vi "UHR-Fleezers Control (host) - 10.6.vi"() -> ()   [LabVIEW 2010] (continued)
          }
        }
      }
      event "Inject Bottom": Value Change {
        n1712 = event-data() -> ("NewVal"=w7676:bool)  [unwired: 6 out]
        n1713 = disable-structure shown="Enabled" {
          disable-tunnel: w7678 -> [_ w7721]
          disable-tunnel: [_ w7720] -> w7677
          disable-tunnel: w7676 -> [_ w7719]
          frame Disabled {
            n1714 = local read "Pump write delay (ms)"() -> (w7680:dbl)
            n1715 = case shown="False" "Inject Bottom" {
              tunnel: w7680 -> [w7687 w7701]
              tunnel: "Chemyx Syringe Pump Serial Port" -> [w7684 w7700]
              frame False {
                n1716 = flat-sequence {
                  tunnel: w7684 -> [w7688]
                  tunnel: [w7688] -> w7685
                  tunnel: w7687 -> [_]
                  tunnel: [w7691] -> w7686
                  tunnel: w7685 -> [w7691]
                  tunnel: w7686 -> [w7692]
                  tunnel: [w7692] -> w7682
                  tunnel: [w7694] -> w7683
                  tunnel: w7682 -> [w7694]
                  tunnel: w7683 -> [w7696]
                  frame #0 {
                    n1717 = call "Write to pump.vi"("string"="enter pump3", "VISA resource name"=w7688) -> ()  [unwired: 1 out]
                  }
                  frame #1 {
                    n1718 = local read "Pump pause delay (ms)"() -> (w7690:u32)
                    n1719 = Wait (ms)(milliseconds to wait=w7690) -> ()  [unwired: 1 out]
                  }
                  frame #2 {
                    n1720 = call "Write to pump.vi"("string"="stop", "VISA resource name"=w7692) -> ()  [unwired: 1 out]
                  }
                  frame #3 {
                    n1721 = Wait (ms)(milliseconds to wait=u32 0) -> ()  [unwired: 1 out]
                  }
                  frame #4 {
                    n1722 = call "Write to pump.vi"("string"="stop", "VISA resource name"=w7696) -> ()  [unwired: 1 out]
                  }
                }
              }
              frame True {
                n1723 = flat-sequence {
                  tunnel: w7700 -> [w7710]
                  tunnel: w7701 -> [w7705]
                  tunnel: w7701 -> [w7712]
                  tunnel: w7700 -> [w7713]
                  tunnel: [w7713] -> w7698
                  tunnel: [w7716] -> w7699
                  tunnel: w7698 -> [w7716]
                  tunnel: w7699 -> [w7717]
                  frame #0 {
                    n1724 = local read "All Pump Parameters"() -> (w7704:T5)
                    n1725 = Unbundle By Name(w7704) -> ("Pump 3"=w7711:T51)
                    n1726 = call "Set pump parameters.vi"("Pump write delay (ms)"=w7705, "Volume (uL)"="Ch 3 Inject Volume (uL)", "Rate (uL/h)"="Ch 3 Inject Rate (ul/h)", "Units"=4.0, "Pump #"=3.0, "Pump Parameters In"=w7711, "VISA resource name"=w7710) -> ("Pump Parameters Out"=w7703:T51)  [unwired: 3 in]
                    n1727 = Bundle By Name(cluster=w7704, "Pump 3"=w7703) -> (w7702:T5)
                    n1728 = local write "All Pump Parameters"(w7702) -> ()
                  }
                  frame #1 {
                    n1729 = Wait (ms)(milliseconds to wait=w7712) -> ()  [unwired: 1 out]
                  }
                  frame #2 {
                    n1730 = call "Write to pump.vi"("string"="start", "VISA resource name"=w7713) -> ()  [unwired: 1 out]
                  }
                  frame #3 {
                    n1731 = Wait (ms)(milliseconds to wait=u32 500) -> ()  [unwired: 1 out]
                  }
                  frame #4 {
                    n1732 = call "Write to pump.vi"("string"="start", "VISA resource name"=w7717) -> ()  [unwired: 1 out]
                  }
                }
              }
            }
          }
          frame Enabled {
            n1733 = call "hamilton_controller.vi"("error in"=w7721, "Open?"=w7719, "valve"=enum16{"A", "B", "C", "D", "ALL"}."B", "action"=T17."MOVE VALVE") -> ("error out"=w7720:errorcluster)  [unwired: 7 in]
          }
        }
      }
      event "Inject Pump 2": Value Change {
        n1734 = event-data() -> ("NewVal"=w7724:bool)  [unwired: 6 out]
        n1735 = disable-structure shown="Enabled" {
          disable-tunnel: w7726 -> [_ w7749]
          disable-tunnel: [_ w7748] -> w7725
          disable-tunnel: w7724 -> [_ w7747]
          frame Disabled {
            n1736 = local read "Pump write delay (ms)"() -> (w7729:dbl)
            n1737 = flat-sequence {
              tunnel: w7727 -> [w7742]
              tunnel: w7729 -> [w7738]
              tunnel: "Inject Pump 2" -> [_]
              tunnel: w7729 -> [w7744]
              tunnel: w7727 -> [w7745]
              frame #0 {
                n1738 = local read "All Pump Parameters"() -> (w7737:T5)
                n1739 = Multiply(x=60.0, y="Flush Center Ch Rate (ul/m)") -> (x*y=w7734:dbl)
                n1740 = Unbundle By Name(w7737) -> ("Pump 2"=w7743:T51)
                n1741 = call "Set pump parameters.vi"("Pump write delay (ms)"=w7738, "Volume (uL)"="Flush Center Ch Volume (uL)", "Rate (uL/h)"=w7734, "Units"=3.0, "Pump #"=2.0, "Pump Parameters In"=w7743, "VISA resource name"=w7742) -> ("Pump Parameters Out"=w7736:T51)  [unwired: 3 in]
                n1742 = Bundle By Name(cluster=w7737, "Pump 2"=w7736) -> (w7735:T5)
                n1743 = local write "All Pump Parameters"(w7735) -> ()
                n1744 = Add(x="Flush Center Ch Volume (uL)", y="Total Volume\nFlushed (uL)") -> (x+y=w7731:dbl)
                n1745 = local write "Total Volume\nFlushed (uL)"(w7731) -> ()
              }
              frame #1 {
                n1746 = Wait (ms)(milliseconds to wait=w7744) -> ()  [unwired: 1 out]
              }
              frame #2 {
                n1747 = call "Write to pump.vi"("string"="start", "VISA resource name"=w7745) -> ()  [unwired: 1 out]
              }
            }
            n1748 = local read "Chemyx Syringe Pump Serial Port"() -> (w7727:refnum<visa-resource-name>)
          }
          frame Enabled {
            n1749 = call "hamilton_controller.vi"("error in"=w7749, "Open?"=w7747, "valve"=enum16{"A", "B", "C", "D", "ALL"}."B", "action"=T17."MOVE VALVE") -> ("error out"=w7748:errorcluster)  [unwired: 7 in]
          }
        }
      }
      event "Sample Channel Flow": Value Change {
        n1750 = event-data() -> ()  [unwired: 7 out]
        n1751 = call "hamilton_controller.vi"("error in"=w7753, "Open?"="Sample Channel Flow", "valve"=enum16{"A", "B", "C", "D", "ALL"}."C", "action"=T17."MOVE VALVE") -> ("error out"=w7752:errorcluster)  [unwired: 7 in]
      }
      event "Flip Green Filter": Value Change {
        n1752 = event-data() -> ()  [unwired: 7 out]
        n1753 = Not(x="Flip Green Filter") -> (.not. x?=w7757:bool)
        n1754 = local write "Flip Green Filter"(w7757) -> ()
        n1755 = flat-sequence {
          tunnel: w7765 -> [w7770]
          tunnel: w7764 -> [w7769]
          tunnel: [w7767] -> w7762
          tunnel: [w7766] -> w7761
          tunnel: [w7810] -> w7760
          tunnel: w7762 -> [w7810]
          tunnel: [w7809] -> w7759
          tunnel: w7761 -> [w7809]
          tunnel: w7760 -> [w7814]
          tunnel: w7759 -> [w7813]
          tunnel: [w7812] -> w7763
          frame #0 {
            n1756 = xnode "Read/Write Control"("FPGA VI Reference In"=w7770, "error in"=w7769, "Green Filter Flipper"=TRUE) -> ("FPGA VI Reference Out"=w7767:T20, "error out"=w7766:errorcluster)
          }
          frame #1 {
            n1757 = Wait (ms)(milliseconds to wait=u32 100) -> ()  [unwired: 1 out]
          }
          frame #2 {
            n1758 = xnode "Read/Write Control"("FPGA VI Reference In"=w7814, "error in"=w7813, "Green Filter Flipper"=FALSE) -> ("error out"=w7812:errorcluster)  [unwired: 1 out]
          }
        }
      }
      event "Pump 1 contents", "Pump 3 contents": Value Change {
        n1759 = event-data() -> ()  [unwired: 7 out]
        n1760 = local read "Pump 1 contents"() -> (→"Pump 1 cont disp":string)
        n1761 = local read "Pump 3 contents"() -> (→"Pump 3 cont disp":string)
      }
      event "Reset Trap Pos. FB": Value Change {
        n1762 = event-data() -> ()  [unwired: 7 out]
        n1763 = xnode "Read/Write Control"("FPGA VI Reference In"=w7858, "error in"=w7857, "Trap Pos. FB Reset"="Reset Trap Pos. FB") -> ()  [unwired: 2 out]
      }
      event "Trap Pos. FB ON": Value Change {
        n1764 = event-data() -> ()  [unwired: 7 out]
        n1765 = xnode "Read/Write Control"("FPGA VI Reference In"=w7899, "error in"=w7898, "Force feedback"="Trap Pos. FB ON") -> ()  [unwired: 2 out]
      }
      event "Trap Pos. FB Range", "Trap Pos. FB Gains", "Trap Pos. FB Mult Factor", "Trap Pos. FB Offset Factor", "Trap Pos FB Negate Action", "Trap Pos FB Monitor\nT1 or T2": Value Change {
        n1766 = event-data() -> ()  [unwired: 7 out]
        n1767 = xnode "Read/Write Control"("FPGA VI Reference In"=w7946, "error in"=w7945, "Trap Pos. FB Range"="Trap Pos. FB Range", "Trap Pos. FB Gains"="Trap Pos. FB Gains", "Trap Pos. FB Mult Factor"="Trap Pos. FB Mult Factor", "Trap Pos. FB Offset Factor"="Trap Pos. FB Offset Factor", "Trap Pos FB Negate Action"="Trap Pos FB Negate Action", "Trap Pos FB Monitor T1 or T2"="Trap Pos FB Monitor\nT1 or T2", "AI1 X Scale"="Trap Pos. AI1 X Pre-scale") -> ()  [unwired: 2 out]
      }
      event "Trap Pos FB SP": Value Change {
        n1768 = event-data() -> ()  [unwired: 7 out]
        n1769 = xnode "Read/Write Control"("FPGA VI Reference In"=w8134, "error in"=w8133, "Trap Pos. FB SP"="Trap Pos FB SP") -> ()  [unwired: 2 out]
      }
      event "Set SP to Reading": Value Change {
        n1770 = event-data() -> ()  [unwired: 7 out]
        n1771 = local read "Trap Pos FB Monitor\nT1 or T2"() -> (w8187:bool)
        n1772 = local read "Trap X AI1 (DMA)"() -> (w8190:T13)
        n1773 = local read "Trap X (AI1)"() -> (w8193:T10)
        n1774 = Unbundle By Name(w8193) -> ("Trap 1"=w8192:fxp<+/-,16,1>, "Trap 2"=w8191:fxp<+/-,16,1>)
        n1775 = Unbundle By Name(w8190) -> ("Set 1"=w8189:fxp<+/-,16,1>, "Set 2"=w8188:fxp<+/-,16,1>)
        n1776 = Select(t=w8192, s=w8187, f=w8191) -> (s? t:f=w8186:fxp<+/-,16,1>)
        n1777 = Select(t=w8189, s=w8187, f=w8188) -> (s? t:f=w8185:fxp<+/-,16,1>)
        n1778 = Not(x="Set SP Using...") -> (.not. x?=w8180:bool)
        n1779 = Select(t=w8186, s=w8180, f=w8185) -> (s? t:f=w8181:fxp<+/-,16,1>)
        n1780 = xnode "Read/Write Control"("FPGA VI Reference In"=w8183, "error in"=w8182, "Trap Pos. FB SP"=w8181) -> ()  [unwired: 2 out]
        n1781 = local write "Trap Pos FB SP"(w8181) -> ()
      }
      event "Trap Pos. FB Out Scale 2^n": Value Change {
        n1782 = event-data() -> ()  [unwired: 7 out]
        n1783 = Scale By Power Of 2(n="Trap Pos. FB Out Scale 2^n", x=ext 1.0) -> (x*2^n=w8240:ext)
        n1784 = property on="Trap Pos. FB Mult Factor" class="DigNum (strict)"("Val(Sgnl)"=w8240) -> ()  [unwired: 2 in, 2 out]
      }
      event "Trap Pos FB Int Count": Value Change {
        n1785 = event-data() -> ()  [unwired: 7 out]
        n1786 = xnode "Read/Write Control"("FPGA VI Reference In"=w8245, "error in"=w8244, "Trap Pos FB Int Count"="Trap Pos FB Int Count") -> ()  [unwired: 2 out]
      }
    }
    "error out 2" <- w4492
    n1787 = node-c288() -> ()  [unwired: 1 in, 1 out]
  }
  n1788 = timed-loop "Run Scripts, including: stage motion" {
    timing: w74 -> [_]
    timing-out: [_] -> w73
    tunnel: w18 -> [_]
    stop <- w8284 stop-if-true
    n1789 = node-c288() -> ()  [unwired: 1 in, 1 out]
    n1790 = event shown="[15] \"Take Detection Laser\nImage\": Value Change" {
      selector: _ -> [_ _ _ _ _ _ _ _ _ _ _ _ _ _ _ _ _]
      dyn-events: _ -> [_ _ _ _ _ _ _ _ _ _ _ _ _ _ _ _ _]
      timeout: 50 -> [_ _ _ _ _ _ _ _ _ _ _ _ _ _ _ _ _]
      tunnel: ["Set Position" "Move to Position" "Move Cap. 1 (DNA Right)" _ "Move Cap. 2 (ADig Left)" _ "Cal/Data Acq. Spot" "Dump Beads" "Dip for Protein" _ _ "Got ADig bead" "Got DNA bead" "Take Stepping Data" _ "Take Detection Laser\nImage" _] -> _
      tunnel: [_ _ _ _ _ _ _ _ _ _ _ _ _ _ _ _ w8671] -> w8284
      event "Set Position", "Set Position 2", "Set Position 3", "Set Position 4", "Set Position 5", "Set Position 1": Value Change {
        n1791 = event-data() -> ()  [unwired: 1 in, 5 out]
        n1792 = Build Array("Set Position 1", "Set Position 2", "Set Position 3", "Set Position 4", "Set Position 5") -> (w8303:bool[])
        n1793 = Boolean Array To Number(Boolean array=w8303) -> (number=w8302:u32)
        n1794 = Logarithm Base 2(1:w8302) -> (0:w8294:dbl)
        n1795 = call "CONEX_FUNCTIONAL_GLOBAL.vi"("Command"=T23."GET POS") -> ("Current Position"=w8287:dbl[])  [unwired: 8 in, 2 out]
        n1796 = Decrement(x="Position") -> (x-1=w8292:dbl)
        n1797 = Greater Or Equal?(x=w8294, y=0.0) -> (x >= y?=w8295:bool)
        n1798 = Select(t=w8294, s=w8295, f=w8292) -> (s? t:f=w8291:dbl)
        n1799 = Increment(x=w8291) -> (x+1=w8290:dbl)
        n1800 = Build Array (concatenate)(w8290, w8287) -> (w8289:dbl[])
        n1801 = Replace Array Subset(array="Saved Stage Positions", new element=w8289, index (row)=w8291) -> (w8304:dbl[][])  [unwired: 1 in]
        n1802 = local write "Saved Stage Positions"(w8304) -> ()
      }
      event "Move to Position": Value Change {
        n1803 = event-data() -> ()  [unwired: 1 in, 5 out]
        n1804 = flat-sequence {
          frame #0 {
            n1805 = local read "Position"() -> (w8319:dbl)
            n1806 = local read "Saved Stage Positions"() -> (w8317:dbl[][])
            n1807 = Decrement(x=w8319) -> (x-1=w8316:dbl)
            n1808 = Array Subset(array=w8317, index (row)=w8316, length (row)=1 ("length"), index (col)=1 ("index"), length (col)=3 ("length")) -> (w8313:dbl[][])
            n1809 = Reshape Array(w8313, 3 ("dimension size")) -> (w8309:dbl[])
            n1810 = local write "Stage Moving"(TRUE ("Stage Moving")) -> ()
            n1811 = call "CONEX_FUNCTIONAL_GLOBAL.vi"("Axis"=enum16{"X", "Y", "Z", "XY", "XZ", "YZ", "XYZ"}."XYZ", "Position"=w8309, "Command"=T23."ABS MOVE") -> ()  [unwired: 6 in, 3 out]
          }
          frame #1 {
            n1812 = call <vilib>:"Beep.vi"() -> ()  [unwired: 3 in, 9 out]
            n1813 = local write "Stage Moving"(FALSE ("Stage Moving")) -> ()
          }
        }
      }
      event "Move Cap. 1 (DNA Right)": Value Change {
        n1814 = event-data() -> ()  [unwired: 1 in, 5 out]
        n1815 = local write "Move Cap. 1 (DNA Right)"(FALSE ("Move Cap. 1 (DNA Right)")) -> ()
        n1816 = flat-sequence {
          tunnel: ["Cap 1 Samp Flow ON"] -> w8322
          tunnel: w8322 -> [w8341]
          tunnel: [w8341] -> w8321
          tunnel: w8321 -> [w8342]
          frame #0 {
            n1817 = local read "Saved Stage Positions"() -> (w8335:dbl[][])
            n1818 = Array Subset(array=w8335, index (row)=0 ("index"), length (row)=1 ("length"), index (col)=1 ("index"), length (col)=3 ("length")) -> (w8332:dbl[][])
            n1819 = Reshape Array(w8332, 3 ("dimension size")) -> (w8326:dbl[])
            n1820 = case shown="True" "Cap 1 Samp Flow ON" {
              frame False {
              }
              frame True {
                n1821 = call "hamilton_controller.vi"("Open?"=TRUE, "valve"=enum16{"A", "B", "C", "D", "ALL"}."C", "action"=T17."MOVE VALVE") -> ()  [unwired: 8 in, 1 out]
              }
            }
            n1822 = call "CONEX_FUNCTIONAL_GLOBAL.vi"("Axis"=enum16{"X", "Y", "Z", "XY", "XZ", "YZ", "XYZ"}."XYZ", "Position"=w8326, "Command"=T23."ABS MOVE") -> ()  [unwired: 6 in, 3 out]
            n1823 = local write "Stage Moving"(TRUE ("Stage Moving")) -> ()
          }
          frame #1 {
            n1824 = call "motor_done_moving.vi"("wait at least (s)"=2.0) -> ()  [unwired: 11 in]
          }
          frame #2 {
            n1825 = local write "Stage Moving"(FALSE ("Stage Moving")) -> ()
            n1826 = case shown="True" w8342 {
              frame False {
              }
              frame True {
                n1827 = call "hamilton_controller.vi"("Open?"=FALSE, "valve"=enum16{"A", "B", "C", "D", "ALL"}."C", "action"=T17."MOVE VALVE") -> ()  [unwired: 8 in, 1 out]
              }
            }
            n1828 = case shown="True" TRUE {
              tunnel: "Cap 1 T ON" -> [w8351 w8352]
              frame False {
                n1829 = property on="Trap 1 (ON/OFF)" class="Bool (strict)"("Val(Sgnl)"=w8351) -> ()  [unwired: 2 in, 2 out]
              }
              frame True {
                n1830 = property on="Trap 2 (ON/OFF)" class="Bool (strict)"("Val(Sgnl)"=w8352) -> ()  [unwired: 2 in, 2 out]
              }
            }
            n1831 = call <vilib>:"Beep.vi"() -> ()  [unwired: 3 in, 9 out]
            n1832 = case shown="True" "Cap 1 Flow ON" {
              frame False {
              }
              frame True {
                n1833 = property on="Inject Top" class="Bool (strict)"("Val(Sgnl)"=TRUE ("Value (Signaling)")) -> ()  [unwired: 2 in, 2 out]
              }
            }
          }
        }
      }
      event Timeout {
        n1834 = event-data() -> ()  [unwired: 1 in, 2 out]
      }
      event "Move Cap. 2 (ADig Left)": Value Change {
        n1835 = event-data() -> ()  [unwired: 1 in, 5 out]
        n1836 = local write "Move Cap. 2 (ADig Left)"(FALSE ("Move Cap. 2 (ADig Left)")) -> ()
        n1837 = flat-sequence {
          tunnel: ["Cap 2 Samp Flow ON"] -> w8354
          tunnel: w8354 -> [w8373]
          tunnel: [w8373] -> w8353
          tunnel: w8353 -> [w8374]
          frame #0 {
            n1838 = local read "Saved Stage Positions"() -> (w8367:dbl[][])
            n1839 = case shown="True" "Cap 2 Samp Flow ON" {
              frame False {
              }
              frame True {
                n1840 = call "hamilton_controller.vi"("Open?"=TRUE, "valve"=enum16{"A", "B", "C", "D", "ALL"}."C", "action"=T17."MOVE VALVE") -> ()  [unwired: 8 in, 1 out]
              }
            }
            n1841 = Array Subset(array=w8367, index (row)=1 ("index"), length (row)=1 ("length"), index (col)=1 ("index"), length (col)=3 ("length")) -> (w8364:dbl[][])
            n1842 = Reshape Array(w8364, 3 ("dimension size")) -> (w8358:dbl[])
            n1843 = local write "Stage Moving"(TRUE ("Stage Moving")) -> ()
            n1844 = call "CONEX_FUNCTIONAL_GLOBAL.vi"("Axis"=enum16{"X", "Y", "Z", "XY", "XZ", "YZ", "XYZ"}."XYZ", "Position"=w8358, "Command"=T23."ABS MOVE") -> ()  [unwired: 6 in, 3 out]
          }
          frame #1 {
            n1845 = call "motor_done_moving.vi"("wait at least (s)"=2.0) -> ()  [unwired: 11 in]
          }
          frame #2 {
            n1846 = local write "Stage Moving"(FALSE ("Stage Moving")) -> ()
            n1847 = case shown="True" TRUE {
              tunnel: "Cap 2 T ON" -> [w8383 w8384]
              frame False {
                n1848 = property on="Trap 2 (ON/OFF)" class="Bool (strict)"("Val(Sgnl)"=w8383) -> ()  [unwired: 2 in, 2 out]
              }
              frame True {
                n1849 = property on="Trap 1 (ON/OFF)" class="Bool (strict)"("Val(Sgnl)"=w8384) -> ()  [unwired: 2 in, 2 out]
              }
            }
            n1850 = call <vilib>:"Beep.vi"() -> ()  [unwired: 3 in, 9 out]
            n1851 = case shown="True" w8374 {
              frame False {
              }
              frame True {
                n1852 = call "hamilton_controller.vi"("Open?"=FALSE, "valve"=enum16{"A", "B", "C", "D", "ALL"}."C", "action"=T17."MOVE VALVE") -> ()  [unwired: 8 in, 1 out]
              }
            }
            n1853 = case shown="True" "Cap 2 Flow ON" {
              frame False {
              }
              frame True {
                n1854 = property on="Inject Bottom" class="Bool (strict)"("Val(Sgnl)"=TRUE ("Value (Signaling)")) -> ()  [unwired: 2 in, 2 out]
              }
            }
          }
        }
      }
      event "+z", "-z": Value Change {
        n1855 = event-data() -> ()  [unwired: 1 in, 5 out]
        n1856 = flat-sequence {
          frame #0 {
            w8386 = 0.0 ("element")
            n1857 = Divide(x="z nudge increment (um)", y=1000.0) -> (x/y=w8399:dbl)
            n1858 = Boolean To (0,1)(Boolean="+z") -> (0, 1=w8392:i16)
            n1859 = Boolean To (0,1)(Boolean="-z") -> (0, 1=w8393:i16)
            n1860 = Multiply(x=w8392, y=w8399) -> (x*y=w8396:dbl)
            n1861 = Multiply(x=w8393, y=w8399) -> (x*y=w8394:dbl)
            n1862 = Negate(x=w8394) -> (-x=w8395:dbl)
            n1863 = Add(x=w8396, y=w8395) -> (x+y=w8387:dbl)
            n1864 = Build Array(w8386, w8386, w8387) -> (w8385:dbl[])
            n1865 = call "CONEX_FUNCTIONAL_GLOBAL.vi"("Axis"=enum16{"X", "Y", "Z", "XY", "XZ", "YZ", "XYZ"}."Z", "Position"=w8385, "Command"=T23."REL MOVE") -> ()  [unwired: 6 in, 3 out]
            n1866 = local write "Stage Moving"(TRUE ("Stage Moving")) -> ()
          }
          frame #1 {
            n1867 = local write "Stage Moving"(FALSE ("Stage Moving")) -> ()
            n1868 = call <vilib>:"Beep.vi"() -> ()  [unwired: 3 in, 9 out]
          }
        }
      }
      event "Cal/Data Acq. Spot": Value Change {
        # "CHANGE FISH FOR TETHER BACK\nTO TRUE VALUE HERE."
        n1869 = event-data() -> ()  [unwired: 1 in, 5 out]
        n1870 = flat-sequence {
          tunnel: ["Cal @ (MHz)"] -> w8402
          tunnel: w8402 -> [w8425]
          tunnel: w8402 -> [w8446]
          frame #0 {
            n1871 = local read "Saved Stage Positions"() -> (w8410:dbl[][])
            n1872 = Array Subset(array=w8410, index (row)=2 ("index"), length (row)=1 ("length"), index (col)=1 ("index"), length (col)=3 ("length")) -> (w8413:dbl[][])
            n1873 = Reshape Array(w8413, 3 ("dimension size")) -> (w8406:dbl[])
            n1874 = local write "Stage Moving"(TRUE ("Stage Moving")) -> ()
            n1875 = call "CONEX_FUNCTIONAL_GLOBAL.vi"("Axis"=enum16{"X", "Y", "Z", "XY", "XZ", "YZ", "XYZ"}."XYZ", "Position"=w8406, "Command"=T23."ABS MOVE") -> ()  [unwired: 6 in, 3 out]
          }
          frame #1 {
            n1876 = call "motor_done_moving.vi"("wait at least (s)"=2.0) -> ()  [unwired: 11 in]
          }
          frame #2 {
            n1877 = property on="Trap Delta (MHz)" class="DigNum (strict)"("Val(Sgnl)"="Cal @ (MHz)") -> ()  [unwired: 2 in, 2 out]
            n1878 = local write "Stage Moving"(FALSE ("Stage Moving")) -> ()
            n1879 = call <vilib>:"Beep.vi"() -> ()  [unwired: 3 in, 9 out]
          }
          frame #3 {
            n1880 = Wait (ms)(milliseconds to wait=u32 100) -> ()  [unwired: 1 out]
          }
          frame #4 {
            n1881 = property on="Save Calibration" class="Bool (strict)"("Val(Sgnl)"=TRUE ("Value (Signaling)")) -> ()  [unwired: 2 in, 2 out]
          }
          frame #5 {
            n1882 = Wait (ms)(milliseconds to wait=u32 4000) -> ()  [unwired: 1 out]
          }
          frame #6 {
            n1883 = while {
              stop <- w8422 stop-if-true
              n1884 = local read "Saving..."() -> (w8423:bool)
              n1885 = Wait (ms)(milliseconds to wait=u32 100) -> ()  [unwired: 1 out]
              n1886 = Not(x=w8423) -> (.not. x?=w8422:bool)
            }
          }
          frame #7 {
            n1887 = case shown="True" "W/ Offset 1" {
              tunnel: w8425 -> [_ w8427]
              frame False {
              }
              frame True {
                n1888 = stacked-sequence {
                  tunnel: w8427 -> [_ _ _ _ _ _ _ w8444]
                  frame #0 {
                    n1889 = property on="Trap Delta (MHz)" class="DigNum (strict)"("Val(Sgnl)"="Offset 1 Start (MHz)") -> ()  [unwired: 2 in, 2 out]
                    n1890 = Replace Array Subset(array=u32[] [0] ("Index Values"), new element="Offset 1 Set", index=0) -> (w8428:u32[])
                    n1891 = property on="Saved AOD Raster Scan Parameter Sets" class="Arr (strict)"("Index Values"=w8428) -> ()  [unwired: 2 in, 2 out]
                  }
                  frame #1 {
                    n1892 = Wait (ms)(milliseconds to wait=u32 200) -> ()  [unwired: 1 out]
                  }
                  frame #2 {
                    n1893 = property on="Load parameters" class="Bool (strict)"("Val(Sgnl)"=TRUE ("Value (Signaling)")) -> ()  [unwired: 2 in, 2 out]
                  }
                  frame #3 {
                    n1894 = Wait (ms)(milliseconds to wait=u32 200) -> ()  [unwired: 1 out]
                  }
                  frame #4 {
                    n1895 = property on="Trap Raster Scan" class="Bool (strict)"("Val(Sgnl)"=TRUE ("Value (Signaling)")) -> ()  [unwired: 2 in, 2 out]
                  }
                  frame #5 {
                    n1896 = Wait (ms)(milliseconds to wait=u32 2000) -> ()  [unwired: 1 out]
                  }
                  frame #6 {
                    n1897 = while {
                      stop <- w8441 stop-if-true
                      n1898 = local read "Raster Scanning..."() -> (w8443:bool)
                      n1899 = local read "Saving..."() -> (w8439:bool)
                      n1900 = Wait (ms)(milliseconds to wait=u32 100) -> ()  [unwired: 1 out]
                      n1901 = Not(x=w8439) -> (.not. x?=w8438:bool)
                      n1902 = Not(x=w8443) -> (.not. x?=w8440:bool)
                      n1903 = And(x=w8440, y=w8438) -> (x .and. y?=w8441:bool)
                    }
                  }
                  frame #7 {
                    n1904 = property on="Trap Delta (MHz)" class="DigNum (strict)"("Val(Sgnl)"=w8444) -> ()  [unwired: 2 in, 2 out]
                  }
                }
              }
            }
          }
          frame #8 {
            n1905 = local read "Save ave N"() -> (w8445:dbl)
            n1906 = case shown="True" "W/ Offset 2" {
              tunnel: w8446 -> [_ w8452]
              tunnel: w8445 -> [_ w8451]
              frame False {
                n1907 = Multiply(x="Cal read wait (s)", y=u32 1000 ("milliseconds to wait")) -> (x*y=w8449:u32)
                n1908 = Wait (ms)(milliseconds to wait=w8449) -> ()  [unwired: 1 out]
              }
              frame True {
                n1909 = stacked-sequence {
                  tunnel: w8452 -> [_ _ _ _ _ _ _ _ _ w8473 _ _]
                  tunnel: w8451 -> [_ _ _ _ _ _ _ _ _ w8471 _ _]
                  frame #0 {
                    n1910 = property on="Save ave N" class="DigNum (strict)"("Val(Sgnl)"=1.0 ("Value (Signaling)")) -> ()  [unwired: 2 in, 2 out]
                  }
                  frame #1 {
                    n1911 = Wait (ms)(milliseconds to wait=u32 500) -> ()  [unwired: 1 out]
                  }
                  frame #2 {
                    n1912 = property on="Trap Delta (MHz)" class="DigNum (strict)"("Val(Sgnl)"="Offset 2 Start (MHz)") -> ()  [unwired: 2 in, 2 out]
                    n1913 = Replace Array Subset(array=u32[] [0] ("Index Values"), new element="Offset 2 Set", index=0) -> (w8457:u32[])
                    n1914 = property on="Saved AOD Raster Scan Parameter Sets" class="Arr (strict)"("Index Values"=w8457) -> ()  [unwired: 2 in, 2 out]
                  }
                  frame #3 {
                    n1915 = Wait (ms)(milliseconds to wait=u32 500) -> ()  [unwired: 1 out]
                  }
                  frame #4 {
                    n1916 = property on="Load parameters" class="Bool (strict)"("Val(Sgnl)"=TRUE ("Value (Signaling)")) -> ()  [unwired: 2 in, 2 out]
                  }
                  frame #5 {
                    n1917 = Wait (ms)(milliseconds to wait=u32 500) -> ()  [unwired: 1 out]
                  }
                  frame #6 {
                    n1918 = property on="Trap Raster Scan" class="Bool (strict)"("Val(Sgnl)"=TRUE ("Value (Signaling)")) -> ()  [unwired: 2 in, 2 out]
                  }
                  frame #7 {
                    n1919 = Wait (ms)(milliseconds to wait=u32 2000) -> ()  [unwired: 1 out]
                  }
                  frame #8 {
                    n1920 = while {
                      stop <- w8466 stop-if-true
                      n1921 = local read "Raster Scanning..."() -> (w8469:bool)
                      n1922 = local read "Saving..."() -> (w8467:bool)
                      n1923 = Wait (ms)(milliseconds to wait=u32 100) -> ()  [unwired: 1 out]
                      n1924 = Not(x=w8467) -> (.not. x?=w8465:bool)
                      n1925 = Not(x=w8469) -> (.not. x?=w8468:bool)
                      n1926 = And(x=w8468, y=w8465) -> (x .and. y?=w8466:bool)
                    }
                  }
                  frame #9 {
                    n1927 = property on="Trap Delta (MHz)" class="DigNum (strict)"("Val(Sgnl)"=w8473) -> ()  [unwired: 2 in, 2 out]
                    n1928 = property on="Saved AOD Raster Scan Parameter Sets" class="Arr (strict)"("Index Values"=u32[] [0]) -> ()  [unwired: 2 in, 2 out]
                    n1929 = property on="Save ave N" class="DigNum (strict)"("Val(Sgnl)"=w8471) -> ()  [unwired: 2 in, 2 out]
                  }
                  frame #10 {
                    n1930 = Wait (ms)(milliseconds to wait=u32 500) -> ()  [unwired: 1 out]
                  }
                  frame #11 {
                    n1931 = property on="Load parameters" class="Bool (strict)"("Val(Sgnl)"=TRUE ("Value (Signaling)")) -> ()  [unwired: 2 in, 2 out]
                  }
                }
              }
            }
          }
          frame #9 {
            n1932 = property on="Read Cal" class="Bool (strict)"("Val(Sgnl)"=TRUE ("Value (Signaling)")) -> ()  [unwired: 2 in, 2 out]
          }
          frame #10 {
            n1933 = Wait (ms)(milliseconds to wait=u32 500) -> ()  [unwired: 1 out]
          }
          frame #11 {
            n1934 = property on="Fish for Tether" class="Bool (strict)"("Val(Sgnl)"="fish after calibration?") -> ()  [unwired: 2 in, 2 out]
          }
        }
        n1935 = local write "Cal/Data Acq. Spot"(FALSE ("Cal/Data Acq. Spot")) -> ()
      }
      event "Dump Beads": Value Change {
        # "SCRIPT TO REMOVE BOTH BEADS FROM THE TRAPS. TURNS ON LIGHT WHICH INDICATES THAT STAGE IS MOVING. THEN STOPS SAVING DATA. \nSETS Sample Channel Flow TO TRUE. STOPS INTERLACING GREEN FLUORESCENCE. TURNS OFF Tether INDICATOR BECAUSE WE ARE THROWING IT\nAWAY. SHUTS OFF TRAP POSITION FEEDBACK."
        n1936 = event-data() -> ()  [unwired: 1 in, 5 out]
        n1937 = flat-sequence {
          frame #0 {
            w8481 = FALSE ("Fl. Triggered...")
            w8480 = TRUE ("Stage Moving")
            n1938 = local read "Saving..."() -> (w8482:bool)
            n1939 = local write "Fl. Triggered..."(w8481) -> ()
            n1940 = local write "Stage Moving"(w8480) -> ()
            n1941 = local write "Tether"(w8481) -> ()
            n1942 = property on="Green Laser ON/Interlacing" class="Bool (strict)"("Val(Sgnl)"=w8481) -> ()  [unwired: 2 in, 2 out]
            n1943 = property on="Trap Pos. FB ON" class="Bool (strict)"("Val(Sgnl)"=w8481) -> ()  [unwired: 2 in, 2 out]
            n1944 = property on="Sample Channel Flow" class="Bool (strict)"("Val(Sgnl)"=w8480) -> ()  [unwired: 2 in, 2 out]
            n1945 = local write "Stop Saving"(w8482) -> ()
          }
          frame #1 {
            # "MOVES TO THE DUMP BEADS POSITION"
            n1946 = local read "Saved Stage Positions"() -> (w8486:dbl[][])
            n1947 = Array Subset(array=w8486, index (row)=3 ("index"), length (row)=1 ("length"), index (col)=1 ("index"), length (col)=3 ("length")) -> (w8489:dbl[][])
            n1948 = Reshape Array(w8489, 3 ("dimension size")) -> (w8484:dbl[])
            n1949 = call "CONEX_FUNCTIONAL_GLOBAL.vi"("Axis"=enum16{"X", "Y", "Z", "XY", "XZ", "YZ", "XYZ"}."XYZ", "Position"=w8484, "Command"=T23."ABS MOVE") -> ()  [unwired: 6 in, 3 out]
          }
          frame #2 {
            n1950 = call "motor_done_moving.vi"("wait at least (s)"=2.0) -> ()  [unwired: 11 in]
          }
          frame #3 {
            w8494 = FALSE ("Value (Signaling)")
            # "TURNS TRAPS OFF SO THAT\nBEADS REMAIN AT DUMP \nBEADS POSITION"
            n1951 = property on="Trap 1 (ON/OFF)" class="Bool (strict)"("Val(Sgnl)"=w8494) -> ()  [unwired: 2 in, 2 out]
            n1952 = property on="Trap 2 (ON/OFF)" class="Bool (strict)"("Val(Sgnl)"=w8494) -> ()  [unwired: 2 in, 2 out]
            n1953 = call <vilib>:"Beep.vi"() -> ()  [unwired: 3 in, 9 out]
          }
          frame #4 {
            # "MOVES STAGE BACK TO THE\nANTIDIG CAPILARY BY CALLING\nTHE Move Cap. 2 SCRIPT"
            n1954 = property on="Move Cap. 2 (ADig Left)" class="Bool (strict)"("Val(Sgnl)"=TRUE ("Value (Signaling)")) -> ()  [unwired: 2 in, 2 out]
          }
        }
      }
      event "Dip for Protein": Value Change {
        n1955 = event-data() -> ()  [unwired: 1 in, 5 out]
        n1956 = flat-sequence {
          frame #0 {
            n1957 = case shown="True" "Move Trap Before?" {
              frame False {
              }
              frame True {
                n1958 = property on="Trap Delta (MHz)" class="DigNum (strict)"("Val(Sgnl)"="Dip Trap Delta 1 (MHz)") -> ()  [unwired: 2 in, 2 out]
              }
            }
          }
          frame #1 {
            n1959 = local read "Saved Stage Positions"() -> (w8502:dbl[][])
            n1960 = Array Subset(array=w8502, index (row)=4 ("index"), length (row)=1 ("length"), index (col)=1 ("index"), length (col)=3 ("length")) -> (w8505:dbl[][])
            n1961 = Reshape Array(w8505, 3 ("dimension size")) -> (w8500:dbl[])
            n1962 = call "CONEX_FUNCTIONAL_GLOBAL.vi"("Axis"=enum16{"X", "Y", "Z", "XY", "XZ", "YZ", "XYZ"}."XYZ", "Position"=w8500, "Command"=T23."ABS MOVE") -> ()  [unwired: 6 in, 3 out]
          }
          frame #2 {
            n1963 = Multiply(x="Duration (s)", y=1000.0) -> (x*y=w8509:dbl)
            n1964 = Wait (ms)(milliseconds to wait=w8509) -> ()  [unwired: 1 out]
          }
          frame #3 {
            n1965 = local read "Saved Stage Positions"() -> (w8515:dbl[][])
            n1966 = Array Subset(array=w8515, index (row)=2 ("index"), length (row)=1 ("length"), index (col)=1 ("index"), length (col)=3 ("length")) -> (w8518:dbl[][])
            n1967 = Reshape Array(w8518, 3 ("dimension size")) -> (w8513:dbl[])
            n1968 = call "CONEX_FUNCTIONAL_GLOBAL.vi"("Axis"=enum16{"X", "Y", "Z", "XY", "XZ", "YZ", "XYZ"}."XYZ", "Position"=w8513, "Command"=T23."ABS MOVE") -> ()  [unwired: 6 in, 3 out]
          }
          frame #4 {
            n1969 = case shown="True" "Move Trap After?" {
              frame False {
              }
              frame True {
                n1970 = property on="Trap Delta (MHz)" class="DigNum (strict)"("Val(Sgnl)"="Dip Trap Delta 2 (MHz)") -> ()  [unwired: 2 in, 2 out]
              }
            }
          }
          frame #5 {
            n1971 = case shown="True" "Green ON After?" {
              frame False {
              }
              frame True {
                n1972 = property on="Green Laser ON/Interlacing" class="Bool (strict)"("Val(Sgnl)"=TRUE ("Value (Signaling)")) -> ()  [unwired: 2 in, 2 out]
              }
            }
          }
          frame #6 {
            n1973 = Wait (ms)(milliseconds to wait=u32 500) -> ()  [unwired: 1 out]
          }
          frame #7 {
            n1974 = case shown="True" "Save Data After?" {
              frame False {
              }
              frame True {
                n1975 = property on="Start Saving" class="Bool (strict)"("Val(Sgnl)"=TRUE ("Value (Signaling)")) -> ()  [unwired: 2 in, 2 out]
              }
            }
          }
        }
      }
      event "Profile": Value Change {
        n1976 = event-data() -> ()  [unwired: 1 in, 5 out]
        n1977 = flat-sequence {
          tunnel: [w8531] -> w8530
          tunnel: w8530 -> [w8535]
          tunnel: [w8534] -> w8529
          tunnel: w8529 -> [w8541]
          frame #0 {
            w8532 = 0.0 ("element")
            n1978 = Build Array(w8532, "Y change (mm)", w8532) -> (w8531:dbl[])
          }
          frame #1 {
            # "move to new position and start saving"
            n1979 = local write "Stage Moving"(TRUE ("Stage Moving")) -> ()
            n1980 = local write "Start Saving"(TRUE ("Start Saving")) -> ()
            n1981 = call "CONEX_FUNCTIONAL_GLOBAL.vi"("Axis"=enum16{"X", "Y", "Z", "XY", "XZ", "YZ", "XYZ"}."Y", "Position"=w8535, "Command"=T23."REL MOVE") -> ()  [unwired: 6 in, 3 out]
            n1982 = Negate(x=w8535) -> (-x=w8534:dbl[])
          }
          frame #2 {
            # "go back to start"
            n1983 = call "CONEX_FUNCTIONAL_GLOBAL.vi"("Axis"=enum16{"X", "Y", "Z", "XY", "XZ", "YZ", "XYZ"}."Y", "Position"=w8541, "Command"=T23."REL MOVE") -> ()  [unwired: 6 in, 3 out]
          }
          frame #3 {
            # "stop saving"
            n1984 = local write "Stop Saving"(TRUE ("Stop Saving")) -> ()
            n1985 = local write "Stage Moving"(FALSE ("Stage Moving")) -> ()
          }
        }
      }
      event "Move to Position 1", "Move to Position 2", "Move to Position 3", "Move to Position 4", "Move to Position 5", "Lower Ch. Cap.": Value Change {
        n1986 = event-data() -> ()  [unwired: 1 in, 5 out]
        n1987 = Or(x="Move to Position 5", y="Lower Ch. Cap.") -> (x .or. y?=w8546:bool)
        n1988 = Build Array("Move to Position 1", "Move to Position 2", "Move to Position 3", "Move to Position 4", w8546) -> (w8549:bool[])
        n1989 = Boolean Array To Number(Boolean array=w8549) -> (number=w8548:u32)
        n1990 = Logarithm Base 2(1:w8548) -> (0:w8547:dbl)
        n1991 = flat-sequence {
          tunnel: w8547 -> [w8559]
          frame #0 {
            n1992 = local read "Saved Stage Positions"() -> (w8564:dbl[][])
            n1993 = Array Subset(array=w8564, index (row)=w8559, length (row)=1 ("length"), index (col)=1 ("index"), length (col)=3 ("length")) -> (w8561:dbl[][])
            n1994 = Reshape Array(w8561, 3 ("dimension size")) -> (w8556:dbl[])
            n1995 = local write "Stage Moving"(TRUE ("Stage Moving")) -> ()
            n1996 = call "CONEX_FUNCTIONAL_GLOBAL.vi"("Axis"=enum16{"X", "Y", "Z", "XY", "XZ", "YZ", "XYZ"}."XYZ", "Position"=w8556, "Command"=T23."ABS MOVE") -> ()  [unwired: 6 in, 3 out]
          }
          frame #1 {
            n1997 = local write "Stage Moving"(FALSE ("Stage Moving")) -> ()
            n1998 = call <vilib>:"Beep.vi"() -> ()  [unwired: 3 in, 9 out]
          }
        }
      }
      event "Got ADig bead": Value Change {
        n1999 = event-data() -> ()  [unwired: 1 in, 5 out]
        n2000 = property on="Move Cap. 1 (DNA Right)" class="Bool (strict)"("Val(Sgnl)"=TRUE ("Value (Signaling)")) -> ()  [unwired: 2 in, 2 out]
        n2001 = property on="Inject Bottom" class="Bool (strict)"("Val(Sgnl)"=FALSE ("Value (Signaling)")) -> ()  [unwired: 2 in, 2 out]
      }
      event "Got DNA bead": Value Change {
        n2002 = event-data() -> ()  [unwired: 1 in, 5 out]
        n2003 = property on="Cal/Data Acq. Spot" class="Bool (strict)"("Val(Sgnl)"=TRUE ("Value (Signaling)")) -> ()  [unwired: 2 in, 2 out]
        n2004 = property on="Inject Top" class="Bool (strict)"("Val(Sgnl)"=FALSE ("Value (Signaling)")) -> ()  [unwired: 2 in, 2 out]
      }
      event "Take Stepping Data": Value Change {
        n2005 = event-data() -> ()  [unwired: 1 in, 5 out]
        n2006 = local read "Save ave N"() -> (w8581:dbl)
        n2007 = flat-sequence {
          tunnel: w8581 -> [w8583]
          tunnel: [w8583] -> w8576
          tunnel: [w8585] -> w8577
          tunnel: w8576 -> [w8585]
          tunnel: [w8587] -> w8578
          tunnel: w8577 -> [w8587]
          tunnel: [w8590] -> w8579
          tunnel: w8578 -> [w8590]
          tunnel: [w8592] -> w8580
          tunnel: w8579 -> [w8592]
          tunnel: [w8594] -> w8574
          tunnel: w8580 -> [w8594]
          tunnel: w8574 -> [w8597]
          tunnel: [w8597] -> w8573
          tunnel: w8573 -> [w8598]
          tunnel: [w8598] -> w8575
          tunnel: w8575 -> [w8604]
          frame #0 {
            n2008 = property on="Save ave N" class="DigNum (strict)"("Val(Sgnl)"="Save ave factor") -> ()  [unwired: 2 in, 2 out]
          }
          frame #1 {
            n2009 = Wait (ms)(milliseconds to wait=u32 100) -> ()  [unwired: 1 out]
          }
          frame #2 {
            n2010 = local read "Offset 2 Start (MHz)"() -> (w8589:dbl)
            n2011 = property on="Saved AOD Raster Scan Parameter Sets" class="Arr (strict)"("Index Values"=u32[] [2]) -> ()  [unwired: 2 in, 2 out]
            n2012 = property on="Trap Delta (MHz)" class="DigNum (strict)"("Val(Sgnl)"=w8589) -> ()  [unwired: 2 in, 2 out]
          }
          frame #3 {
            n2013 = property on="Load parameters" class="Bool (strict)"("Val(Sgnl)"=TRUE ("Value (Signaling)")) -> ()  [unwired: 2 in, 2 out]
          }
          frame #4 {
            n2014 = Wait (ms)(milliseconds to wait=u32 100) -> ()  [unwired: 1 out]
          }
          frame #5 {
            n2015 = property on="Trap Raster Scan" class="Bool (strict)"("Val(Sgnl)"=TRUE ("Value (Signaling)")) -> ()  [unwired: 2 in, 2 out]
          }
          frame #6 {
            n2016 = Wait (ms)(milliseconds to wait=u32 1000) -> ()  [unwired: 1 out]
          }
          frame #7 {
            n2017 = while {
              stop <- w8601 stop-if-true
              n2018 = local read "Raster Scanning..."() -> (w8603:bool)
              n2019 = local read "Saving..."() -> (w8602:bool)
              n2020 = Not(x=w8602) -> (.not. x?=w8599:bool)
              n2021 = Not(x=w8603) -> (.not. x?=w8600:bool)
              n2022 = And(x=w8600, y=w8599) -> (x .and. y?=w8601:bool)
            }
          }
          frame #8 {
            n2023 = property on="Save ave N" class="DigNum (strict)"("Val(Sgnl)"=w8604) -> ()  [unwired: 2 in, 2 out]
          }
        }
      }
      event "Step Size (nm)": Value Change {
        n2024 = event-data() -> ()  [unwired: 1 in, 5 out]
        n2025 = flat-sequence {
          frame #0 {
            n2026 = property on="Saved AOD Raster Scan Parameter Sets" class="Arr (strict)"("Index Values"=u32[] [1]) -> ()  [unwired: 2 in, 2 out]
          }
          frame #1 {
            n2027 = Multiply(x="N Steps", y="Step Size (nm)") -> (x*y=w8606:dbl)
            n2028 = property on="Scan Speed AOD (nm/s) 2" class="DigNum (strict)"("Value"="Step Size (nm)") -> ()  [unwired: 2 in, 2 out]
            n2029 = property on="Step Size AOD (nm) 2" class="DigNum (strict)"("Value"="Step Size (nm)") -> ()  [unwired: 2 in, 2 out]
            n2030 = property on="Scan Range AOD (nm) 2" class="DigNum (strict)"("Value"=w8606) -> ()  [unwired: 2 in, 2 out]
          }
        }
      }
      event "Take Detection Laser\nImage": Value Change {
        n2031 = event-data() -> ()  [unwired: 1 in, 5 out]
        n2032 = flat-sequence {
          tunnel: [w8637] -> w8625
          tunnel: [w8636] -> w8618
          tunnel: [w8635] -> w8610
          tunnel: [w8633] -> w8609
          tunnel: [w8640] -> w8626
          tunnel: w8625 -> [w8640]
          tunnel: [w8639] -> w8619
          tunnel: w8618 -> [w8639]
          tunnel: [w8638] -> w8611
          tunnel: w8610 -> [w8638]
          tunnel: [w8644] -> w8627
          tunnel: w8626 -> [w8644]
          tunnel: [w8643] -> w8620
          tunnel: w8619 -> [w8643]
          tunnel: [w8642] -> w8612
          tunnel: w8611 -> [w8642]
          tunnel: [w8650] -> w8628
          tunnel: w8627 -> [w8650]
          tunnel: [w8649] -> w8621
          tunnel: w8620 -> [w8649]
          tunnel: [w8648] -> w8613
          tunnel: w8612 -> [w8648]
          tunnel: [w8654] -> w8629
          tunnel: w8628 -> [w8654]
          tunnel: [w8653] -> w8622
          tunnel: w8621 -> [w8653]
          tunnel: [w8652] -> w8614
          tunnel: w8613 -> [w8652]
          tunnel: [w8658] -> w8630
          tunnel: w8629 -> [w8658]
          tunnel: [w8657] -> w8623
          tunnel: w8622 -> [w8657]
          tunnel: [w8656] -> w8615
          tunnel: w8614 -> [w8656]
          tunnel: [w8662] -> w8631
          tunnel: w8630 -> [w8662]
          tunnel: [w8661] -> w8624
          tunnel: w8623 -> [w8661]
          tunnel: [w8660] -> w8616
          tunnel: w8615 -> [w8660]
          tunnel: w8631 -> [w8668]
          tunnel: w8624 -> [w8667]
          tunnel: [w8665] -> w8617
          tunnel: w8616 -> [w8665]
          tunnel: w8617 -> [w8670]
          tunnel: w8609 -> [w8669]
          frame #0 {
            n2033 = local read "Green Laser ON/Interlacing"() -> (w8637:bool)
            n2034 = local read "APD Gate"() -> (w8633:enum32{"ON", "OFF", "Interlace"})
            n2035 = local read "Green laser mode"() -> (w8636:enum32{"Laser ON", "Laser OFF", "Interlace"})
            n2036 = local read "Green FB On/Off"() -> (w8635:bool)
            n2037 = property on="APD Gate" class="RadioBtnsControl (strict)"("Val(Sgnl)"=enum32{"ON", "OFF", "Interlace"}."OFF" ("Value (Signaling)")) -> ()  [unwired: 2 in, 2 out]
          }
          frame #1 {
            n2038 = property on="Green FB On/Off" class="Bool (strict)"("Val(Sgnl)"=FALSE ("Value (Signaling)")) -> ()  [unwired: 2 in, 2 out]
          }
          frame #2 {
            n2039 = property on="Green Laser ON/Interlacing" class="Bool (strict)"("Val(Sgnl)"=TRUE ("Value (Signaling)")) -> ()  [unwired: 2 in, 2 out]
            n2040 = property on="Flip Green Filter" class="Bool (strict)"("Val(Sgnl)"=TRUE ("Value (Signaling)")) -> ()  [unwired: 2 in, 2 out]
            n2041 = property on="Green laser mode" class="RadioBtnsControl (strict)"("Val(Sgnl)"=enum32{"Laser ON", "Laser OFF", "Interlace"}."Laser ON" ("Value (Signaling)")) -> ()  [unwired: 2 in, 2 out]
          }
          frame #3 {
            n2042 = Wait (ms)(milliseconds to wait=u32 500) -> ()  [unwired: 1 out]
          }
          frame #4 {
            n2043 = property on="Confocal Image" class="Bool (strict)"("Val(Sgnl)"=TRUE ("Value (Signaling)")) -> ()  [unwired: 2 in, 2 out]
          }
          frame #5 {
            n2044 = Wait (ms)(milliseconds to wait=u32 2000) -> ()  [unwired: 1 out]
          }
          frame #6 {
            n2045 = while {
              stop <- w8663 stop-if-true
              n2046 = local read "Saving..."() -> (w8664:bool)
              n2047 = Not(x=w8664) -> (.not. x?=w8663:bool)
            }
          }
          frame #7 {
            n2048 = property on="Flip Green Filter" class="Bool (strict)"("Val(Sgnl)"=FALSE ("Value (Signaling)")) -> ()  [unwired: 2 in, 2 out]
            n2049 = property on="Green Laser ON/Interlacing" class="Bool (strict)"("Val(Sgnl)"=w8668) -> ()  [unwired: 2 in, 2 out]
            n2050 = property on="Green laser mode" class="RadioBtnsControl (strict)"("Val(Sgnl)"=w8667) -> ()  [unwired: 2 in, 2 out]
          }
          frame #8 {
            n2051 = property on="Green FB On/Off" class="Bool (strict)"("Val(Sgnl)"=w8670) -> ()  [unwired: 2 in, 2 out]
            n2052 = property on="APD Gate" class="RadioBtnsControl (strict)"("Val(Sgnl)"=w8669) -> ()  [unwired: 2 in, 2 out]
          }
        }
      }
      event "Stop All": Value Change {
        n2053 = event-data() -> ()  [unwired: 1 in, 5 out]
        n2054 = local read "Stop All"() -> (w8671:bool)
      }
    }
    n2055 = node-c288() -> ()  [unwired: 1 in, 1 out]
  }
  n2056 = timed-loop "Mouse control: trap position (AOM deflection), set confocal spot from image" {
    tunnel: [w8673] -> w33
    tunnel: w18 -> [w8672]
    timing: w81 -> [_]
    timing-out: [_] -> w80
    stop <- w8673 stop-if-true
    n2057 = node-c288() -> ()  [unwired: 2 out]
    n2058 = event shown="[0] \"Pane\": Mouse Down" {
      selector: _ -> [_ _]
      dyn-events: _ -> [_ _]
      timeout: _ -> [_ _]
      tunnel: w8672 -> [w8676 _]
      event Mouse Down {
        n2059 = event-data() -> ("Time"=w8678:u32, "Coords"=w8677:T7, "Button"=w8679:u16)  [unwired: 6 out]
        n2060 = case shown="3" w8679 {
          tunnel: w8678 -> [_ _ w8782]
          tunnel: w8677 -> [_ w8716 w8780]
          tunnel: w8676 -> [_ _ w8778]
          frame 0, Default {
          }
          frame 1 {
            n2061 = property on="APD 2" class="ImageControl"() -> ("Displayed Image Position"=w8686:cluster{"Left":i32, "Top":i32})  [unwired: 2 in, 2 out]
            n2062 = property on="APD 1" class="ImageControl"() -> ("Displayed Image Position"=w8715:cluster{"Left":i32, "Top":i32})  [unwired: 2 in, 2 out]
            n2063 = property on="Detection Laser X" class="ImageControl"() -> ("Displayed Image Position"=w8712:cluster{"Left":i32, "Top":i32})  [unwired: 2 in, 2 out]
            n2064 = property on="Detection Laser Y" class="ImageControl"() -> ("Displayed Image Position"=w8711:cluster{"Left":i32, "Top":i32})  [unwired: 2 in, 2 out]
            n2065 = property on="APD 2" class="ImageControl"() -> ("Displayed Image Size"=w8685:cluster{"Width":u32, "Height":u32})  [unwired: 2 in, 2 out]
            n2066 = property on="APD 1" class="ImageControl"() -> ("Displayed Image Size"=w8713:cluster{"Width":u32, "Height":u32})  [unwired: 2 in, 2 out]
            n2067 = property on="Detection Laser X" class="ImageControl"() -> ("Displayed Image Size"=w8714:cluster{"Width":u32, "Height":u32})  [unwired: 2 in, 2 out]
            n2068 = property on="Detection Laser Y" class="ImageControl"() -> ("Displayed Image Size"=w8710:cluster{"Width":u32, "Height":u32})  [unwired: 2 in, 2 out]
            n2069 = Unbundle By Name(w8685) -> ("Width"=w8682:u32, "Height"=w8681:u32)
            n2070 = Unbundle By Name(w8686) -> ("Left"=w8684:i32, "Top"=w8683:i32)
            n2071 = Unbundle By Name(w8713) -> ("Width"=w8707:u32, "Height"=w8706:u32)
            n2072 = Unbundle By Name(w8714) -> ("Width"=w8703:u32, "Height"=w8702:u32)
            n2073 = Unbundle By Name(w8710) -> ("Width"=w8699:u32, "Height"=w8698:u32)
            n2074 = Unbundle By Name(w8715) -> ("Left"=w8709:i32, "Top"=w8708:i32)
            n2075 = Unbundle By Name(w8712) -> ("Left"=w8705:i32, "Top"=w8704:i32)
            n2076 = Unbundle By Name(w8711) -> ("Left"=w8701:i32, "Top"=w8700:i32)
            n2077 = Bundle("Left"=w8684, "Top"=w8683, "Width"=w8682, "Height"=w8681) -> (w8680:T52)  [unwired: 1 in]
            n2078 = Bundle("Left"=w8709, "Top"=w8708, "Width"=w8707, "Height"=w8706) -> (w8697:T52)  [unwired: 1 in]
            n2079 = Bundle("Left"=w8705, "Top"=w8704, "Width"=w8703, "Height"=w8702) -> (w8696:T52)  [unwired: 1 in]
            n2080 = Bundle("Left"=w8701, "Top"=w8700, "Width"=w8699, "Height"=w8698) -> (w8695:T52)  [unwired: 1 in]
            n2081 = Build Cluster Array(w8680, w8697, w8696, w8695) -> (w8694:T53)
            n2082 = for {
              tunnel: w8716 -> [w8727]
              tunnel: w8694 -> [w8728] mode=indexing
              shift-right: [w8725] -> w8692
              shift-left: TRUE -> [w8726]
              shift-right: [w8724] -> w8690
              shift-left: _ -> [w8720]
              shift-right: [w8723] -> w8689
              shift-left: _ -> [w8719]
              shift-right: [w8722] -> w8688
              shift-left: _ -> [w8718]
              shift-right: [w8721] -> w8687
              shift-left: _ -> [w8717]
              n2083 = case shown="True" w8726 {
                selector: w8726 -> [w8733 _]
                tunnel: w8728 -> [_ w8742]
                tunnel: w8727 -> [_ w8740]
                tunnel: [w8733 w8738] -> w8725
                tunnel: [w8732 w8737] -> w8724
                tunnel: [w8731 w8736] -> w8723
                tunnel: [w8730 w8735] -> w8722
                tunnel: [w8729 w8734] -> w8721
                tunnel: w8720 -> [w8732 _]
                tunnel: w8719 -> [w8731 _]
                tunnel: w8718 -> [w8730 _]
                tunnel: w8717 -> [w8729 _]
                frame False {
                }
                frame True {
                  n2084 = Unbundle(w8742) -> (w8741:T52)
                  n2085 = call "isclickinwindow.vi"("Image Param"=w8741, "Point32"=w8740) -> ("4 Y"=w8734:i32, "3 Height"=w8735:i32, "2 X"=w8736:i32, "1 Width"=w8737:i32, "In image?"=w8739:bool)  [unwired: 1 in]
                  n2086 = Not(x=w8739) -> (.not. x?=w8738:bool)
                }
              }
            }
            n2087 = Not(x=w8692) -> (.not. x?=w8691:bool)
            n2088 = case shown="True" w8691 {
              tunnel: w8689 -> [_ w8755]
              tunnel: w8687 -> [_ w8754]
              tunnel: w8690 -> [_ w8753]
              tunnel: w8688 -> [_ w8752]
              frame False {
              }
              frame True {
                w8748 = FALSE ("Get Point")
                n2089 = local read "Scan lines (y)"() -> (w8757:u64)
                n2090 = local read "Actual MCL Inc (V)"() -> (w8749:dbl)
                n2091 = local read "Scan steps (MCL)"() -> (w8756:u64)
                n2092 = Divide "Y Pix/step"(x=w8752, y=w8757) -> (x/y=w8764:dbl)
                n2093 = Divide "Y V/pix"(x=w8749, y=w8764) -> (x/y=w8763:dbl)
                n2094 = Divide "Y half step offset"(x=w8749, y=2.0) -> (x/y=w8765:dbl)